vi "UHR-Fleezers Control (host) - Avogadro v1.vi"() -> ()   [LabVIEW 2014] (continued)
      }
      event "Green Laser ON/OFF", "Red Laser ON/OFF", "Blue Laser ON/OFF": Value Change {
        # "This loop shouldn't be initialized.  The main 'laser ON' settings should dominate and set the others."
        n1323 = event-data() -> ()  [unwired: 7 out]
        n1324 = property on="Red Laser ON" class="Bool (strict)"("Val(Sgnl)"="Red Laser ON/OFF") -> ()  [unwired: 2 in, 2 out]
        n1325 = property on="Blue Laser ON" class="Bool (strict)"("Val(Sgnl)"="Blue Laser ON/OFF") -> ()  [unwired: 2 in, 2 out]
        n1326 = property on="Green Laser ON" class="Bool (strict)"("Val(Sgnl)"="Green Laser ON/OFF") -> ()  [unwired: 2 in, 2 out]
      }
      event "Laser interlacing mode", "Green Laser ON", "Red Laser ON", "Blue Laser ON": Value Change {
        n1327 = event-data() -> ()  [unwired: 7 out]
        n1328 = local write "Green Laser ON/OFF"("Green Laser ON") -> ()
        n1329 = local write "Blue Laser ON/OFF"("Blue Laser ON") -> ()
        n1330 = local write "Red Laser ON/OFF"("Red Laser ON") -> ()
        n1331 = case shown="False" "Green Laser ON" {
          tunnel: "Laser interlacing mode" -> [_ w2112]
          tunnel: [enum32{"Laser ON", "Laser OFF", "Interlace"}."Laser OFF" ("Green laser mode") w2112] -> w2088
          tunnel: [FALSE w2108] -> w2087
          frame False {
          }
          frame True {
            n1332 = local read "Green FB On/Off"() -> (w2109:bool)
            n1333 = Equal?(x=w2112, y=enum32{"Laser ON", "Laser OFF", "Interlace"}."Interlace") -> (x = y?=w2110:bool)
            n1334 = And(x=w2110, y=w2109) -> (x .and. y?=w2108:bool)
          }
        }
        n1335 = case shown="True" "Red Laser ON" {
          tunnel: "Laser interlacing mode" -> [_ w2105]
          tunnel: [enum32{"Laser ON", "Laser OFF", "Interlace"}."Laser OFF" ("Green laser mode") w2105] -> w2084
          tunnel: [FALSE w2101] -> w2083
          frame False {
          }
          frame True {
            n1336 = local read "Red FB On/Off"() -> (w2102:bool)
            n1337 = Equal?(x=w2105, y=enum32{"Laser ON", "Laser OFF", "Interlace"}."Interlace") -> (x = y?=w2103:bool)
            n1338 = And(x=w2103, y=w2102) -> (x .and. y?=w2101:bool)
          }
        }
        n1339 = case shown="True" "Blue Laser ON" {
          tunnel: "Laser interlacing mode" -> [_ w2096]
          tunnel: [enum32{"Laser ON", "Laser OFF", "Interlace"}."Laser OFF" ("Green laser mode") w2096] -> w2080
          tunnel: [FALSE w2094] -> w2079
          frame False {
          }
          frame True {
            n1340 = local read "Blue FB On/Off"() -> (w2095:bool)
            n1341 = Equal?(x=w2096, y=enum32{"Laser ON", "Laser OFF", "Interlace"}."Interlace") -> (x = y?=w2097:bool)
            n1342 = And(x=w2097, y=w2095) -> (x .and. y?=w2094:bool)
          }
        }
        n1343 = xnode "Read/Write Control"("FPGA VI Reference In"=w2078, "Operating Mode"=w2088, "Operating Mode 2"=w2088, "Green FB On/Off"=w2087, "Red Laser Operating Mode"=w2084, "RI Operating Mode 2"=w2084, "Red FB On/Off"=w2083, "BI Operating Mode (AO)"=w2080, "Blue Laser Operating Mode (D)"=w2080, "Blue FB On/Off"=w2079) -> ("error out"=w2089:errorcluster)  [unwired: 1 in, 1 out]
        n1344 = local read "Red FB On/Off"() -> (w2061:bool)
        n1345 = local read "Green FB On/Off"() -> (w2063:bool)
        n1346 = local read "Green Laser ON"() -> (w2062:bool)
        n1347 = local read "Red Laser ON"() -> (w2060:bool)
        n1348 = And(x=w2061, y=w2060) -> (x .and. y?=w2066:bool)
        n1349 = And(x=w2063, y=w2062) -> (x .and. y?=w2072:bool)
        n1350 = local read "Red laser intensity (V)"() -> (w2065:dbl)
        n1351 = local read "Red FB Setpoint (mV)"() -> (w2064:dbl)
        n1352 = local read "Green FB Setpoint (mV)"() -> (w2075:dbl)
        n1353 = local read "Green laser intensity (V)"() -> (w2077:dbl)
        n1354 = Multiply(x=w2065, y=1000.0) -> (x*y=w2069:dbl)
        n1355 = Subtract(x=w2064, y=5.0) -> (x-y=w2068:dbl)
        n1356 = Multiply(x=w2077, y=1000.0) -> (x*y=w2074:dbl)
        n1357 = Subtract(x=w2075, y=5.0) -> (x-y=w2073:dbl)
        n1358 = Less Or Equal?(x=w2069, y=w2068) -> (x <= y?=w2067:bool)
        n1359 = Less Or Equal?(x=w2074, y=w2073) -> (x <= y?=w2071:bool)
        n1360 = And(x=w2066, y=w2067) -> (x .and. y?=w2056:bool)
        n1361 = And(x=w2072, y=w2071) -> (x .and. y?=w2057:bool)
        n1362 = Or(x=w2057, y=w2056) -> (x .or. y?=w2055:bool)
        n1363 = case shown="True" w2055 {
          frame False {
            n1364 = local write "Laser Intensity Low (bugs to fix)"(FALSE ("Laser Intensity Low")) -> ()
          }
          frame True {
            n1365 = local write "Laser Intensity Low (bugs to fix)"(TRUE ("Laser Intensity Low")) -> ()
          }
        }
      }
      event "Invert laser interlacing": Value Change {
        n1366 = event-data() -> ()  [unwired: 7 out]
        n1367 = xnode "Read/Write Control"("FPGA VI Reference In"=w2113, "Invert GI"="Invert laser interlacing", "Invert GI 2"="Invert laser interlacing", "Invert RI"="Invert laser interlacing", "Invert RI 2"="Invert laser interlacing", "Invert BI (AO)"="Invert laser interlacing", "Invert BI (D)"="Invert laser interlacing") -> ("error out"=w2115:errorcluster)  [unwired: 1 in, 1 out]
      }
      event "Green FB Setpoint (mV)", "Green FB Gains", "Green FB On/Off", "Green Intensity % (FB OFF)", "Green int current ON count adj": Value Change {
        n1368 = event-data() -> ()  [unwired: 7 out]
        n1369 = local read "Green FB Setpoint (mV)"() -> (w2135:dbl)
        n1370 = Multiply(x=w2135, y=3.2767) -> (x*y=w2134:dbl)
        n1371 = local read "Green Intensity % (FB OFF)"() -> (w2138:dbl)
        n1372 = Multiply(x=w2138, y=655.35) -> (x*y=w2139:dbl)
        n1373 = To Unsigned Word Integer(number=w2139) -> (unsigned 16bit integer=w2137:u16)
        n1374 = local read "Green int current ON count adj"() -> (w2141:u32)
        n1375 = local read "Laser interlacing mode"() -> (w2132:enum32{"Laser ON", "Laser OFF", "Interlace"})
        n1376 = local read "Green FB Gains"() -> (w2129:T14)
        n1377 = local read "Green Laser ON"() -> (w2133:bool)
        n1378 = local read "Green FB On/Off"() -> (w2142:bool)
        n1379 = Equal?(x=w2132, y=enum32{"Laser ON", "Laser OFF", "Interlace"}."Interlace") -> (x = y?=w2130:bool)
        n1380 = Unbundle By Name(w2129) -> ("proportional gain (Kc)"=w2128:i16, "integral gain (Kc*Ts/Ti)"=w2127:i16, "derivative gain (Kc*Td/Ts)"=w2126:i16)
        n1381 = Compound Arithmetic op=AND(w2130, w2142, w2133) -> (w2116:bool)
        n1382 = local read "Green FB Setpoint (mV)"() -> (w2120:dbl)
        n1383 = local read "Green laser intensity (V)"() -> (w2123:dbl)
        n1384 = xnode "Read/Write Control"("FPGA VI Reference In"=w2125, "Green FB Setpoint"=w2134, "Green FB On/Off"=w2116, "Current Out"=w2137, "Green int current ON count adj"=w2141, "P3"=w2128, "I3"=w2127, "D3"=w2126) -> ("error out"=w2143:errorcluster)  [unwired: 1 in, 1 out]
        n1385 = Multiply(x=w2123, y=1000.0) -> (x*y=w2119:dbl)
        n1386 = Subtract(x=w2120, y=5.0) -> (x-y=w2118:dbl)
        n1387 = Less Or Equal?(x=w2119, y=w2118) -> (x <= y?=w2117:bool)
        n1388 = And(x=w2116, y=w2117) -> (x .and. y?=w2124:bool)
        n1389 = case shown="True" w2124 {
          frame False {
            n1390 = local write "Laser Intensity Low (bugs to fix)"(FALSE ("Laser Intensity Low")) -> ()
          }
          frame True {
            n1391 = local write "Laser Intensity Low (bugs to fix)"(TRUE ("Laser Intensity Low")) -> ()
          }
        }
      }
      event "Blue FB Setpoint (mV)", "Blue FB Gains", "Blue FB On/Off", "Blue Intensity % (FB OFF)", "Blue int AO ON count adjust": Value Change {
        # "Triggers blue laser serial command"
        # "16 bit analog out"
        n1392 = event-data() -> ()  [unwired: 7 out]
        n1393 = Multiply(x="Blue FB Setpoint (mV)", y=3.2767) -> (x*y=w2163:dbl)
        n1394 = Multiply(x="Blue Intensity % (FB OFF)", y=0.8) -> (x*y=w2146:dbl)
        n1395 = Number To Decimal String(number=w2146) -> (decimal integer string=w2147:string)  [unwired: 1 in]
        n1396 = Multiply(x="Blue Intensity % (FB OFF)", y=655.35) -> (x*y=w2166:dbl)
        n1397 = local write "Blue Laser Power (mW)\n(Constant Power Mode)"(w2147) -> ()
        n1398 = To Unsigned Word Integer(number=w2166) -> (unsigned 16bit integer=w2165:u16)
        n1399 = local read "Laser interlacing mode"() -> (w2161:enum32{"Laser ON", "Laser OFF", "Interlace"})
        n1400 = Unbundle By Name("Blue FB Gains") -> ("proportional gain (Kc)"=w2158:i16, "integral gain (Kc*Ts/Ti)"=w2157:i16, "derivative gain (Kc*Td/Ts)"=w2156:i16)
        n1401 = local read "Blue Laser ON"() -> (w2151:bool)
        n1402 = Equal?(x=w2161, y=enum32{"Laser ON", "Laser OFF", "Interlace"}."Interlace") -> (x = y?=w2159:bool)
        n1403 = Compound Arithmetic op=AND(w2159, "Blue FB On/Off", w2151) -> (w2162:bool)
        n1404 = xnode "Read/Write Control"("FPGA VI Reference In"=w2150, "Blue FB Setpoint"=w2163, "Blue FB On/Off"=w2162, "BI Current Out"=w2165, "Blue current ON count adj (AO)"="Blue int AO ON count adjust", "P5"=w2158, "I5"=w2157, "D5"=w2156) -> ("error out"=w2168:errorcluster)  [unwired: 1 in, 1 out]
      }
      event "Red FB Setpoint (mV)", "Red FB Gains", "Red FB On/Off", "Red Intensity % (FB OFF)": Value Change {
        n1405 = event-data() -> ()  [unwired: 7 out]
        n1406 = local read "Red FB Setpoint (mV)"() -> (w2189:dbl)
        n1407 = Multiply(x=w2189, y=3.2767) -> (x*y=w2188:dbl)
        n1408 = local read "Red Intensity % (FB OFF)"() -> (w2179:dbl)
        n1409 = Multiply(x=w2179, y=655.35) -> (x*y=w2192:dbl)
        n1410 = To Unsigned Word Integer(number=w2192) -> (unsigned 16bit integer=w2191:u16)
        n1411 = local read "Laser interlacing mode"() -> (w2186:enum32{"Laser ON", "Laser OFF", "Interlace"})
        n1412 = local read "Red FB Gains"() -> (w2183:T14)
        n1413 = local read "Red Laser ON"() -> (w2187:bool)
        n1414 = local read "Red FB On/Off"() -> (w2194:bool)
        n1415 = Equal?(x=w2186, y=enum32{"Laser ON", "Laser OFF", "Interlace"}."Interlace") -> (x = y?=w2184:bool)
        n1416 = Unbundle By Name(w2183) -> ("proportional gain (Kc)"=w2182:i16, "integral gain (Kc*Ts/Ti)"=w2181:i16, "derivative gain (Kc*Td/Ts)"=w2180:i16)
        n1417 = Compound Arithmetic op=AND(w2184, w2194, w2187) -> (w2171:bool)
        n1418 = local read "Red laser intensity (V)"() -> (w2170:dbl)
        n1419 = local read "Red FB Setpoint (mV)"() -> (w2169:dbl)
        n1420 = xnode "Read/Write Control"("FPGA VI Reference In"=w2178, "Red FB Setpoint"=w2188, "Red FB On/Off"=w2171, "RI Current Out"=w2191, "P4"=w2182, "I4"=w2181, "D4"=w2180) -> ("error out"=w2195:errorcluster)  [unwired: 1 in, 1 out]
        n1421 = Multiply(x=w2170, y=1000.0) -> (x*y=w2175:dbl)
        n1422 = Subtract(x=w2169, y=5.0) -> (x-y=w2174:dbl)
        n1423 = Less Or Equal?(x=w2175, y=w2174) -> (x <= y?=w2173:bool)
        n1424 = And(x=w2171, y=w2173) -> (x .and. y?=w2172:bool)
        n1425 = case shown="False" w2172 {
          frame False {
            n1426 = local write "Laser Intensity Low (bugs to fix)"(FALSE ("Laser Intensity Low")) -> ()
          }
          frame True {
            n1427 = local write "Laser Intensity Low (bugs to fix)"(TRUE ("Laser Intensity Low")) -> ()
          }
        }
      }
      event "+ phase (APD 1 Gate)", "- phase (APD 1 Gate)", "+ phase (APD 2 Gate)", "- phase (APD 2 Gate)", "+ phase (APD 3 Gate)", "- phase (APD 3 Gate)", "+ phase (APD Acq)", "- phase (APD Acq)": Value Change {
        n1428 = event-data() -> ()  [unwired: 7 out]
        n1429 = local read "Phase Adj. (APD 1 Gate)"() -> (w2218:i16)
        n1430 = Or(x="- phase (APD 1 Gate)", y="+ phase (APD 1 Gate)") -> (x .or. y?=w2220:bool)
        n1431 = Negate(x=w2218) -> (-x=w2225:i16)
        n1432 = Select(t=w2225, s="+ phase (APD 1 Gate)", f=w2218) -> (s? t:f=w2224:i16)
        n1433 = local read "Phase Adj. (APD 2 Gate)"() -> (w2215:i16)
        n1434 = Or(x="- phase (APD 2 Gate)", y="+ phase (APD 2 Gate)") -> (x .or. y?=w2213:bool)
        n1435 = Negate(x=w2215) -> (-x=w2217:i16)
        n1436 = Select(t=w2217, s="+ phase (APD 2 Gate)", f=w2215) -> (s? t:f=w2214:i16)
        n1437 = Negate(x="Phase Adj. (APD 3 Gate)") -> (-x=w2212:i16)
        n1438 = Or(x="- phase (APD 3 Gate)", y="+ phase (APD 3 Gate)") -> (x .or. y?=w2208:bool)
        n1439 = Select(t=w2212, s="+ phase (APD 3 Gate)", f="Phase Adj. (APD 3 Gate)") -> (s? t:f=w2209:i16)
        n1440 = local read "Phase Adj. (APD Acq)"() -> (w2206:i16)
        n1441 = Or(x="- phase (APD Acq)", y="+ phase (APD Acq)") -> (x .or. y?=w2204:bool)
        n1442 = Negate(x=w2206) -> (-x=w2207:i16)
        n1443 = Select(t=w2207, s="+ phase (APD Acq)", f=w2206) -> (s? t:f=w2205:i16)
        n1444 = xnode "Read/Write Control"("FPGA VI Reference In"=w2198, "Phase count adjustment (APD 1 Gate)"=w2224, "Phase count adjustment (APD 2 Gate)"=w2214, "Phase count adjustment (APD 3 Gate)"=w2209, "Phase Count Adjustment (APD Acq)"=w2205) -> ("FPGA VI Reference Out"=w2222:T41, "error out"=w2223:errorcluster)  [unwired: 1 in]
        n1445 = xnode "Read/Write Control"("FPGA VI Reference In"=w2222, "error in"=w2223, "+ phase (APD 1 Gate)"=w2220, "+ phase (APD 2 Gate)"=w2213, "+ phase (APD 3 Gate)"=w2208, "+ phase (APD Acq)"=w2204) -> ("error out"=w2221:errorcluster)  [unwired: 1 out]
      }
      event "Invert APD Gate", "APD Gate ON Count", "APD Gate OFF Count", "APD Gate", "APD Integration Time (s)", "APD AO Scale Factor", "Duty Frequency (ON 1/N cycles)", "Interlace ON count", "Interlace OFF count": Value Change {
        n1446 = event-data() -> ()  [unwired: 7 out]
        n1447 = Add(x="Interlace ON count", y="Interlace OFF count") -> (x+y=w2232:u16)
        n1448 = Add(x="APD Gate ON Count", y="APD Gate OFF Count") -> (x+y=w2243:u16)
        n1449 = Multiply(x="Duty Frequency (ON 1/N cycles)", y=w2232) -> (x*y=w2228:u16)
        "Green AI Count" <- w2228
        "Red AI Count" <- w2228
        "Blue AI Count" <- w2228
        n1450 = Subtract(x=w2228, y="Interlace ON count") -> (x-y=w2231:u16)
        n1451 = Multiply(x=w2243, y="Duty Frequency (ON 1/N cycles)") -> (x*y=w2242:u16)
        n1452 = Subtract(x=w2242, y="APD Gate ON Count") -> (x-y=w2241:u16)
        n1453 = local read "DMA Update Period (s)"() -> (w2244:dbl)
        n1454 = Multiply(x="APD Integration Time (s)", y=40000000.0) -> (x*y=w2248:dbl)
        n1455 = Reciprocal(x="APD Integration Time (s)") -> (1/x=→"APD Acq Rate (Hz)":dbl)
        n1456 = To Unsigned Long Integer(number=w2248) -> (unsigned 32bit integer=w2234:u32)
        "APD Int. Count" <- w2234
        n1457 = local read "Number of APDs"() -> (w2227:u8)
        n1458 = Divide(x=w2244, y="APD Integration Time (s)") -> (x/y=w2246:dbl)
        n1459 = Multiply(x=w2227, y=w2246) -> (x*y=w2245:dbl)
        n1460 = local write "APD Samples/FIFO Acq."(w2246) -> ()
        n1461 = local write "APD Elements/DMA read"(w2245) -> ()
        n1462 = xnode "Read/Write Control"("FPGA VI Reference In"=w2226, "Invert APD Gate"="Invert APD Gate", "APD Gate ON Count"="APD Gate ON Count", "APD Gate OFF Count"=w2241, "APD Acq Rate Count"=w2234, "APD Gate Operating Mode"="APD Gate", "APD AO scale factor"="APD AO Scale Factor", "Green interlace ON count"="Interlace ON count", "Green interlace OFF count"=w2231, "Green interlace ON count 2"="Interlace ON count", "Green interlace OFF count 2"=w2231, "Green FB Count"=w2228, "Red interlace ON count"="Interlace ON count", "Red interlace OFF count"="Interlace OFF count", "Blue ON count (AO)"="Interlace ON count", "Blue OFF count (AO)"="Interlace OFF count", "Blue interlace OFF count (D)"="Interlace OFF count", "Blue interlace ON count (D)"="Interlace ON count") -> ("error out"=w2250:errorcluster)  [unwired: 1 in, 1 out]
      }
      event "Neg. TTrig FPGA": Value Change {
        n1463 = event-data() -> ()  [unwired: 7 out]
        n1464 = xnode "Read/Write Control"("FPGA VI Reference In"=w2251, "TTrig Negate Pos"="Neg. TTrig FPGA") -> ()  [unwired: 1 in, 2 out]
      }
      event "Test ttrig": Value Change {
        n1465 = event-data() -> ()  [unwired: 7 out]
        n1466 = xnode "Read/Write Control"("FPGA VI Reference In"=w2253, "TTrig?"=TRUE) -> ("error out"=w2255:errorcluster)  [unwired: 1 in, 1 out]
      }
      event "Number of F/B Scans (AOD)", "Scan Speed (nm/s)", "Scan BD", "Initial delta (MHz)", "Step Size (nm)", "Scan Range (nm)": Value Change {
        w2319 = 123.0  # AOM cal (nm/MHz)
        n1467 = event-data() -> ()  [unwired: 7 out]
        n1468 = local read "BD 1 Frequency 1 (MHz)"() -> (w2302:dbl)
        n1469 = local read "AOM X Cal (nm/MHz)"() -> (w2294:dbl)
        n1470 = local read "X RF Frequency Limits (MHz)"() -> (w2306:T23)
        n1471 = local read "Y RF Frequency Limits (MHz)"() -> (w2303:T23)
        n1472 = local read "BD 2 Frequency 1 (MHz)"() -> (w2308:dbl)
        n1473 = Negate(x="Scan Range (nm)") -> (-x=w2272:dbl)
        n1474 = Divide(x=w2272, y=w2294) -> (x/y=w2276:dbl)
        n1475 = Select(t=w2306, s="Scan BD", f=w2303) -> (s? t:f=w2305:T23)
        n1476 = Select(t=w2302, s="Scan BD", f=w2308) -> (s? t:f=w2307:dbl)
        n1477 = Unbundle By Name(w2305) -> ("Maximum"=w2314:dbl, "Minimum"=w2313:dbl)
        n1478 = Add(x=w2276, y=w2307) -> (x+y=w2311:dbl)
        n1479 = Divide(x=w2272, y="Step Size (nm)") -> (x/y=w2291:dbl)
        n1480 = Divide(x="Step Size (nm)", y=w2294) -> (x/y=w2300:dbl)
        n1481 = Absolute Value(x=w2291) -> (abs(x)=w2275:dbl)
        n1482 = Sign(1:w2272) -> (0:w2273:dbl)
        n1483 = In Range and Coerce(upper limit=w2314, x=w2311, lower limit=w2313) -> (coerced(x)=w2310:dbl, In Range?=w2312:bool)
        n1484 = To Unsigned Quad Integer(1:w2275) -> (0:w2290:u64)
        "Scan steps (AOD)" <- w2290
        n1485 = call "IR AOM freq to word.vi"("Frequency In (MHz)"=w2300) -> ("Frequency Word Out (double)"=w2297:dbl)
        n1486 = Multiply(x=w2273, y=w2297) -> (x*y=w2274:dbl)
        n1487 = Subtract(x=w2311, y=w2310) -> (x-y=w2309:dbl)
        n1488 = To Quad Integer(1:w2274) -> (0:w2296:i64)
        "Incr. int (AOD)" <- w2296
        n1489 = Subtract(x=w2276, y=w2309) -> (x-y=w2295:dbl)
        "Scan Range (MHz)" <- w2295
        n1490 = Select(t=w2276, s=w2312, f=w2295) -> (s? t:f=w2315:dbl)
        n1491 = Multiply(x=w2295, y=w2294) -> (x*y=w2293:dbl)
        n1492 = Decrement(x=w2290) -> (x-1=w2343:u64)
        n1493 = Negate(x=w2293) -> (-x=w2289:dbl)
        n1494 = local write "Scan Range (nm)"(w2289) -> ()
        n1495 = Divide(x=w2315, y=w2343) -> (x/y=w2299:dbl)
        "Scan Increment (MHz)" <- w2299
        n1496 = call "IR AOM freq to word.vi"("Frequency In (MHz)"=w2299) -> ("Frequency Word Out (double)"=w2298:dbl)
        n1497 = Divide(x="Step Size (nm)", y="Scan Speed (nm/s)") -> (x/y=w2286:dbl)
        n1498 = To Quad Integer(1:w2298) -> ()  [unwired: 1 out]
        n1499 = local read "Number Interlace Sets"() -> (w2270:u8)
        n1500 = local read "AI Count (ticks)"() -> (w2271:u16)
        n1501 = local read "Total Counts (ticks)"() -> (w2269:u16)
        n1502 = local read "# Samples/trap"() -> (w2301:u32)
        n1503 = Multiply(x=w2271, y=w2270) -> (x*y=w2268:u16)
        n1504 = Divide(x=w2269, y=w2268) -> (x/y=w2267:dbl)
        n1505 = Select(t=w2302, s="Scan BD", f=w2308) -> (s? t:f=w2340:dbl)
        "Initial freq. (MHz)" <- w2340
        n1506 = Add(x=w2315, y=w2340) -> (x+y=→"Final freq. (MHz)":dbl)
        n1507 = Divide(x=w2269, y=40000000.0) -> (x/y=w2285:dbl)
        n1508 = Divide(x=w2286, y=w2285) -> (x/y=w2284:dbl)
        n1509 = To Unsigned Quad Integer(1:w2284) -> (0:w2259:u64)
        n1510 = Quotient & Remainder(x=w2259, y=u64 2) -> (x-y*floor(x/y)=w2263:u64)  [unwired: 1 out]
        n1511 = Equal?(x=w2263, y=u64 0) -> (x = y?=w2261:bool)
        n1512 = Decrement(x=w2259) -> (x-1=w2260:u64)
        n1513 = Select(t=w2259, s=w2261, f=w2260) -> (s? t:f=w2258:u64)
        "Cycles/step (AOD)" <- w2258
        n1514 = xnode "Read/Write Control"("FPGA VI Reference In"=w2257, "Scan steps"=w2290, "Number of scans"="Number of F/B Scans (AOD)", "Cycles per step"=w2258, "Scan freq.  increment"=w2296, "Scan BD"="Scan BD") -> ("error out"=w2349:errorcluster)  [unwired: 1 in, 1 out]
        n1515 = Multiply(x=w2290, y=w2258) -> (x*y=w2344:u64)
        n1516 = Multiply(x=w2344, y=u64 2) -> (x*y=w2266:u64)
        n1517 = Multiply(x=w2267, y=w2266) -> (x*y=w2265:dbl)
        "Data points/scan (f/b)" <- w2265
        n1518 = Multiply(x=w2265, y="Number of F/B Scans (AOD)") -> (x*y=w2347:dbl)
        "Data points/scans" <- w2347
        n1519 = Divide(x=w2347, y=w2301) -> (x/y=→"N sets should be saved":dbl)
        n1520 = Multiply(x=w2344, y=w2285) -> (x*y=w2283:dbl)
        "Time/Scan (s) (AOD)" <- w2283
        n1521 = Select(t=w2315, s="Scan BD", f=0.0) -> (s? t:f=w2341:dbl)
        n1522 = Select(t=0.0, s="Scan BD", f=w2315) -> (s? t:f=w2337:dbl)
        n1523 = local read "BD 2 Frequency 2 (MHz)"() -> (w2333:dbl)
        n1524 = local read "BD 1 Frequency 2 (MHz)"() -> (w2336:dbl)
        n1525 = Add(x=w2337, y=w2308) -> (x+y=w2334:dbl)
        n1526 = Add(x=w2302, y=w2341) -> (x+y=w2335:dbl)
        n1527 = Multiply(x=w2283, y=2.0) -> (x*y=w2282:dbl)
        n1528 = Multiply(x=w2282, y="Number of F/B Scans (AOD)") -> (x*y=w2279:dbl)
        n1529 = Divide(x=w2279, y=60.0) -> (x/y=→"Time to Finish All (min)":dbl)
        n1530 = Add(x="Trap 2 Bead Size (nm)", y="Trap 1 Bead Size (nm)") -> (x+y=w2323:dbl)
        n1531 = Divide(x=w2323, y=2.0) -> (x/y=w2317:dbl)
        n1532 = local read "Initial delta (MHz)"() -> (w2320:dbl)
        n1533 = Subtract(x=w2334, y=w2333) -> (x-y=w2331:dbl)
        n1534 = Subtract(x=w2335, y=w2336) -> (x-y=w2332:dbl)
        n1535 = Square(x=w2331) -> (x^2=w2330:dbl)
        n1536 = Square(x=w2332) -> (x^2=w2329:dbl)
        n1537 = Add(x=w2329, y=w2330) -> (x+y=w2328:dbl)
        n1538 = Square Root(x=w2328) -> (sqrt(x)=w2327:dbl)
        "Final delta (MHz)" <- w2327
        n1539 = Multiply(x=w2319, y=w2327) -> (x*y=w2326:dbl)
        n1540 = Multiply(x=w2320, y=w2319) -> (x*y=w2318:dbl)
        n1541 = Subtract(x=w2318, y=w2317) -> (x-y=→"Initial sep (nm)":dbl)
        n1542 = Subtract(x=w2326, y=w2317) -> (x-y=→"Final sep (nm)":dbl)
      }
      event "Freq or Amp switch first", "Swap F1 and F2", "Freq switch delay", "Amp switch delay": Value Change {
        n1543 = event-data() -> ()  [unwired: 7 out]
        n1544 = local read "Amp switch delay"() -> (w2351:u16)
        n1545 = local read "Swap F1 and F2"() -> (w2352:bool)
        n1546 = xnode "Read/Write Control"("FPGA VI Reference In"=w2350, "Swap F1 and F2"=w2352, "Amp switch delay"=w2351) -> ("error out"=w2353:errorcluster)  [unwired: 1 in, 1 out]
      }
      event "Scan steps (MCL)", "Number of scans (MCL)", "Scan Range (V)\n(of steps)", "2D or 1D Scan", "N APD Samp/step", "Fast Scan Dir", "Continuous MCL Scanning", "Scan lines (y)": Value Change {
        w2356 = 32767.0 ("y")
        n1547 = event-data() -> ()  [unwired: 7 out]
        n1548 = Select(t="Scan lines (y)", s="2D or 1D Scan", f="Number of scans (MCL)") -> (s? t:f=w2361:u64)
        n1549 = Decrement(x="Scan steps (MCL)") -> (x-1=w2377:u64)
        n1550 = Divide(x="Scan Range (V)\n(of steps)", y=w2377) -> (x/y=w2376:dbl)
        "Desired Scan Incr (V)" <- w2376
        n1551 = local read "APD Integration Time (s)"() -> (w2369:dbl)
        n1552 = Multiply(x=w2376, y=w2356) -> (x*y=w2385:dbl)
        n1553 = Divide(x=w2385, y=10.0) -> (x/y=w2375:dbl)
        "Desired incr (int)" <- w2375
        n1554 = local read "Update Count (MCL)"() -> (w2381:u32)
        n1555 = Round Toward -Infinity(1:w2375) -> (0:w2384:dbl)
        n1556 = To Word Integer(number=w2384) -> (16bit integer=w2359:i16)
        "Actual Incr. int (MCL)" <- w2359
        n1557 = Multiply(x=w2369, y=40000000.0) -> (x*y=w2382:dbl)
        n1558 = Divide(x=w2382, y=w2381) -> (x/y=w2380:dbl)
        n1559 = Multiply(x=i16 10, y=w2359) -> (x*y=w2357:i16)
        n1560 = Multiply(x="N APD Samp/step", y=w2380) -> (x*y=w2379:dbl)
        "Cycles/step (MCL)" <- w2379
        n1561 = Divide(x=w2357, y=w2356) -> (x/y=→"Actual MCL Inc (V)":dbl)
        n1562 = Multiply(x="N APD Samp/step", y="Scan steps (MCL)") -> (x*y=w2371:dbl)
        n1563 = local read "APD Samples/FIFO Acq."() -> (w2368:dbl)
        n1564 = Multiply(x=w2371, y=u64 2) -> (x*y=w2370:dbl)
        "Data points/scan (f+b)" <- w2370
        n1565 = Multiply(x=w2370, y=w2361) -> (x*y=w2388:dbl)
        "Data points/scans (MCL)" <- w2388
        n1566 = Multiply(x=w2369, y=w2370) -> (x*y=w2362:dbl)
        "Time/f+b scan (s) (MCL)" <- w2362
        n1567 = Divide(x=w2388, y=w2368) -> (x/y=→"N sets should be saved (MCL)":dbl)
        n1568 = Multiply(x=w2362, y=w2361) -> (x*y=→"Total Time (s)":dbl)
        n1569 = Not(x="Fast Scan Dir") -> (.not. x?=w2366:bool)
        n1570 = xnode "Read/Write Control"("FPGA VI Reference In"=w2354, "Scan steps (MCL)"="Scan steps (MCL)", "Number of scans (MCL)"=w2361, "Cycles per step (MCL)"=w2379, "Scan freq.  increment (MCL)"=w2359, "1D or 2D Scan?"="2D or 1D Scan", "MCL Scan Axis"=w2366, "Cont. Scan (MCL)"="Continuous MCL Scanning") -> ("error out"=w2390:errorcluster)  [unwired: 1 in, 1 out]
      }
      event "Read Cal": Value Change {
        w2411 = T45."big-endian, network order" ("byte order (0:big-endian, network order)")
        n1571 = event-data() -> ()  [unwired: 7 out]
        n1572 = local read "Save file name"() -> (w2443:path)
        n1573 = Strip Path(path=w2443) -> (stripped path=w2442:path)  [unwired: 1 out]
        n1574 = Path To String(path=w2442) -> (string=w2435:string)
        n1575 = Concatenate Strings(w2435, "\\current.cal" ("string")) -> (w2440:string)
        n1576 = String To Path(string=w2440) -> (path=w2439:path)
        n1577 = Open/Create/Replace File(file path (use dialog)=w2439, operation (0:open)=T44."open", access (0:read/write)=enum16{"read/write", "read-only", "write-only"}."read-only") -> (refnum out=w2446:refnum<file>, error out=w2438:errorcluster)  [unwired: 1 in, 3 out]
        n1578 = Concatenate Strings(w2435, "\\current.off" ("string")) -> (w2433:string)
        n1579 = Deny Access(4:w2438, 7:w2446) -> (0:w2412:errorcluster, 3:w2407:refnum<file>)  [unwired: 1 out]
        n1580 = String To Path(string=w2433) -> (path=w2430:path)
        n1581 = local write "Read Cal"(FALSE ("Read Cal")) -> ()
        n1582 = Open/Create/Replace File(file path (use dialog)=w2430, operation (0:open)=T44."open", access (0:read/write)=enum16{"read/write", "read-only", "write-only"}."read-only") -> (refnum out=w2429:refnum<file>)  [unwired: 1 in, 4 out]
        n1583 = Deny Access(7:w2429) -> (3:w2428:refnum<file>)  [unwired: 1 in, 2 out]
        n1584 = Read from Binary File(5:0.0, 9:w2411, 10:-1 ("count (1)"), 11:w2428) -> (2:w2423:dbl[], 3:w2421:refnum<file>)  [unwired: 1 in, 3 out]
        n1585 = Close File(refnum=w2421) -> ()  [unwired: 1 in, 2 out]
        n1586 = Index Array(array=w2423, index=0) -> (element=→"Offset file step size":dbl)
        n1587 = Array Subset(array=w2423, index=1) -> (w2420:dbl[])  [unwired: 1 in]
        n1588 = Decimate 1D Array(w2420) -> (w2416:dbl[], w2415:dbl[])  [unwired: 1 out]
        n1589 = Build Array("T1 calibration", "T2 calibration", "T3 calibration") -> (w2403:T47)
        n1590 = for {
          N: 3 ("count (1)") -> [_]
          tunnel: w2411 -> [w2464]
          shift-right: [w2462] -> w2409
          shift-left: w2412 -> [w2465]
          shift-right: [w2461] -> w2408
          shift-left: w2407 -> [w2460]
          tunnel: w2403 -> [w2459] mode=indexing
          tunnel: [w2452] -> w2402 mode=indexing
          i -> [w2453]
          w2451 = 1000.0
          n1591 = Read from Binary File(5:0.0, 8:w2465, 9:w2464, 10:6 ("count (1)"), 11:w2460) -> (0:w2462:errorcluster, 2:w2467:dbl[], 3:w2461:refnum<file>)  [unwired: 2 out]
          n1592 = Array To Cluster(array=w2467) -> (cluster=w2458:T48)
          n1593 = Unbundle(w2458) -> ("[0]"=w2457:dbl, "[1]"=w2456:dbl, "[2]"=w2449:dbl, "[3]"=w2455:dbl, "[4]"=w2454:dbl, "[5]"=w2450:dbl)
          n1594 = Multiply(x=w2451, y=w2450) -> (x*y=w2447:dbl)
          n1595 = Multiply(x=w2451, y=w2449) -> (x*y=w2448:dbl)
          n1596 = Bundle By Name(cluster=w2459, "alpha_x (nm/V)"=w2457, "kappa_x (pN/nm)"=w2456, "offset_x (mV)"=w2448, "alpha_y (nm/V)"=w2455, "kappa_y (pN/nm)"=w2454, "offset_y (mV)"=w2447) -> (w2452:T9)
          n1597 = case shown="2" w2453 {
            tunnel: w2452 -> [w2468 w2469 w2470]
            frame 0, Default {
              n1598 = local write "T1 calibration"(w2468) -> ()
            }
            frame 1 {
              n1599 = local write "T2 calibration"(w2469) -> ()
            }
            frame 2 {
              n1600 = local write "T3 calibration"(w2470) -> ()
            }
          }
        }
        n1601 = Bundle By Name(cluster="Offset Values", "Trap 1X offset"=w2416, "Trap 2X offset"=w2415) -> (w2418:T20)
        n1602 = local write "Offset Values"(w2418) -> ()
        n1603 = Index Array(array=w2402, index=1) -> (element=w2399:T9)
        n1604 = Index Array(array=w2402, index=0) -> (element=w2398:T9)
        n1605 = Unbundle By Name(w2399) -> ("alpha_x (nm/V)"=w2397:dbl, "kappa_x (pN/nm)"=w2396:dbl)
        n1606 = Unbundle By Name(w2398) -> ("alpha_x (nm/V)"=w2395:dbl, "kappa_x (pN/nm)"=w2394:dbl)
        n1607 = Close File(refnum=w2408, error in=w2409) -> (error out=→"Read cal error":errorcluster)  [unwired: 1 out]
        n1608 = Multiply(x=w2397, y=w2396) -> (x*y=w2393:dbl)
        n1609 = Multiply(x=w2395, y=w2394) -> (x*y=w2392:dbl)
        n1610 = Divide(x=w2393, y=w2392) -> (x/y=w2391:dbl)
        n1611 = property on="B factor" class="DigNum (strict)"("Val(Sgnl)"=w2391) -> ()  [unwired: 2 in, 2 out]
        n1612 = Multiply(x=w2415, y=w2391) -> (x*y=w2417:dbl[])
        n1613 = Subtract(x=w2416, y=w2417) -> (x-y=w2413:dbl[])
        n1614 = case shown="True" "Auto read offset correction" {
          tunnel: w2413 -> [_ w2471]
          frame False {
          }
          frame True {
            n1615 = property on="Setpoint offset\ncorrection values" class="Arr (strict)"("Val(Sgnl)"=w2471) -> ()  [unwired: 2 in, 2 out]
          }
        }
      }
      event "Abort MCL Scan": Value Change {
        n1616 = event-data() -> ()  [unwired: 7 out]
        n1617 = local write "MCL Scanning"(FALSE ("MCL Scanning")) -> ()
        n1618 = xnode "Read/Write Control"("FPGA VI Reference In"=w2472, "Abort scan (MCL)"="Abort MCL Scan") -> ("error out"=w2475:errorcluster)  [unwired: 1 in, 1 out]
      }
      event "Update Count (MCL)": Value Change {
        n1619 = event-data() -> ()  [unwired: 7 out]
        n1620 = xnode "Read/Write Control"("FPGA VI Reference In"=w2476, "MCL count"="Update Count (MCL)") -> ("error out"=w2478:errorcluster)  [unwired: 1 in, 1 out]
      }
      event "+ phase (MCL)", "- phase (MCL)": Value Change {
        n1621 = event-data() -> ()  [unwired: 7 out]
        n1622 = Or(x="- phase (MCL)", y="+ phase (MCL)") -> (x .or. y?=w2482:bool)
        n1623 = Negate(x="Phase adjust (MCL)") -> (-x=w2488:i16)
        n1624 = Select(t=w2488, s="+ phase (MCL)", f="Phase adjust (MCL)") -> (s? t:f=w2486:i16)
        n1625 = xnode "Read/Write Control"("FPGA VI Reference In"=w2479, "Phase count adjustment (MCL)"=w2486) -> ("FPGA VI Reference Out"=w2483:T41, "error out"=w2484:errorcluster)  [unwired: 1 in]
        n1626 = xnode "Read/Write Control"("FPGA VI Reference In"=w2483, "error in"=w2484, "+ phase (MCL)"=w2482) -> ("error out"=w2481:errorcluster)  [unwired: 1 out]
      }
      event "Abort AOD Scan": Value Change {
        n1627 = event-data() -> ()  [unwired: 7 out]
        n1628 = xnode "Read/Write Control"("FPGA VI Reference In"=w2489, "Abort scan"="Abort AOD Scan") -> ("error out"=w2491:errorcluster)  [unwired: 1 in, 1 out]
      }
      event "Continuous AOD Scanning": Value Change {
        n1629 = event-data() -> ()  [unwired: 7 out]
        n1630 = xnode "Read/Write Control"("FPGA VI Reference In"=w2492, "Cont. Scan"="Continuous AOD Scanning") -> ("error out"=w2494:errorcluster)  [unwired: 1 in, 1 out]
      }
      event "Index": Value Change {
        n1631 = event-data() -> ()  [unwired: 7 out]
        n1632 = call "Create new save file.vi"("Insert"="", "Ext"=".dat" ("string"), "Index In"="Index") -> ("Path Out"=→"Save file name":path, "Index Out"=w2495:dbl)
        "Save index" <- w2495
        n1633 = local write "Index"(w2495) -> ()
      }
      event "AO1", "AO2": Value Change {
        w2509 = 10.0 ("y")
        w2508 = 32767.0 ("y")
        n1634 = event-data() -> ()  [unwired: 7 out]
        n1635 = local read "AO2"() -> (w2507:dbl)
        n1636 = local read "AO1"() -> (w2504:dbl)
        n1637 = Multiply(x=w2504, y=w2508) -> (x*y=w2503:dbl)
        n1638 = Multiply(x=w2507, y=w2508) -> (x*y=w2506:dbl)
        n1639 = Divide(x=w2503, y=w2509) -> (x/y=w2502:dbl)
        n1640 = Divide(x=w2506, y=w2509) -> (x/y=w2505:dbl)
        n1641 = To Word Integer(number=w2502) -> (16bit integer=w2510:i16)
        n1642 = To Word Integer(number=w2505) -> (16bit integer=w2511:i16)
        n1643 = xnode "Read/Write Control"("FPGA VI Reference In"=w2500, "AO1 (Y)"=w2510, "AO2 (X)"=w2511) -> ("error out"=w2501:errorcluster)  [unwired: 1 in, 1 out]
      }
      event "Inject Pump 1": Value Change {
        n1644 = event-data() -> ()  [unwired: 7 out]
        n1645 = disable-structure shown="Disabled" {
          disable-tunnel: w2512 -> [w2513 _]
          frame Disabled {
            n1646 = local read "Use Harvard pumps\nfor beads (else Chemyx)"() -> (w2514:bool)
            n1647 = case shown="True" w2514 {
              tunnel: "Inject Pump 1" -> [w2518 w2559]
              tunnel: w2513 -> [_ w2560]
              frame False {
                n1648 = local read "Pump write delay (ms)"() -> (w2517:dbl)
                n1649 = local read "Chemyx Syringe Pump Serial Port"() -> (w2516:refnum<visa-resource-name>)
                n1650 = case shown="True" w2518 {
                  tunnel: w2517 -> [w2524 w2538]
                  tunnel: w2516 -> [w2521 w2537]
                  frame False {
                    n1651 = flat-sequence {
                      tunnel: w2521 -> [w2525]
                      tunnel: [w2525] -> w2522
                      tunnel: w2524 -> [_]
                      tunnel: [w2528] -> w2523
                      tunnel: w2522 -> [w2528]
                      tunnel: w2523 -> [w2529]
                      tunnel: [w2529] -> w2519
                      tunnel: [w2531] -> w2520
                      tunnel: w2519 -> [w2531]
                      tunnel: w2520 -> [w2533]
                      frame #0 {
                        n1652 = call "Write to pump.vi"("string"="enter pump1", "VISA resource name"=w2525) -> ()  [unwired: 1 out]
                      }
                      frame #1 {
                        n1653 = Wait (ms)(milliseconds to wait="Pump pause delay (ms)") -> ()  [unwired: 1 out]
                      }
                      frame #2 {
                        n1654 = call "Write to pump.vi"("string"="stop", "VISA resource name"=w2529) -> ()  [unwired: 1 out]
                      }
                      frame #3 {
                        n1655 = Wait (ms)(milliseconds to wait=u32 500) -> ()  [unwired: 1 out]
                      }
                      frame #4 {
                        n1656 = call "Write to pump.vi"("string"="stop", "VISA resource name"=w2533) -> ()  [unwired: 1 out]
                      }
                    }
                  }
                  frame True {
                    n1657 = flat-sequence {
                      tunnel: w2537 -> [w2547]
                      tunnel: w2538 -> [w2542]
                      tunnel: w2538 -> [w2549]
                      tunnel: w2537 -> [w2550]
                      tunnel: [w2550] -> w2535
                      tunnel: [w2552] -> w2536
                      tunnel: w2535 -> [w2552]
                      tunnel: w2536 -> [w2554]
                      frame #0 {
                        n1658 = local read "All Pump Parameters"() -> (w2541:T10)
                        n1659 = Unbundle By Name(w2541) -> ("Pump 1"=w2548:T49)
                        n1660 = call "Set pump parameters.vi"("Pump write delay (ms)"=w2542, "Volume (uL)"="Ch 1 Inject Volume (uL)", "Rate (uL/h)"="Ch 1 Inject Rate (ul/h)", "Units"=4.0, "Pump #"=1.0, "Pump Parameters In"=w2548, "VISA resource name"=w2547) -> ("Pump Parameters Out"=w2540:T49)  [unwired: 3 in]
                        n1661 = Bundle By Name(cluster=w2541, "Pump 1"=w2540) -> (w2539:T10)
                        n1662 = local write "All Pump Parameters"(w2539) -> ()
                      }
                      frame #1 {
                        n1663 = Wait (ms)(milliseconds to wait=w2549) -> ()  [unwired: 1 out]
                      }
                      frame #2 {
                        n1664 = call "Write to pump.vi"("string"="start", "VISA resource name"=w2550) -> ()  [unwired: 1 out]
                      }
                      frame #3 {
                        n1665 = Wait (ms)(milliseconds to wait=u32 500) -> ()  [unwired: 1 out]
                      }
                      frame #4 {
                        n1666 = call "Write to pump.vi"("string"="start", "VISA resource name"=w2554) -> ()  [unwired: 1 out]
                      }
                    }
                  }
                }
              }
              frame True {
                n1667 = case shown="False" w2559 {
                  tunnel: w2560 -> [w2572 w2582]
                  frame False {
                    n1668 = flat-sequence {
                      tunnel: w2572 -> [w2574]
                      frame #0 {
                        n1669 = local write "Flushing P1"(FALSE ("Flushing P1")) -> ()
                        n1670 = Concatenate Strings("stop" ("string"), "\r") -> (w2576:string)
                        n1671 = VISA Write(VISA resource name=w2574, write buffer=w2576) -> ()  [unwired: 1 in, 3 out]
                      }
                      frame #1 {
                        n1672 = property on="Clear Volume P1" class="Bool (strict)"("Val(Sgnl)"=TRUE ("Value (Signaling)")) -> ()  [unwired: 2 in, 2 out]
                      }
                    }
                  }
                  frame True {
                    n1673 = local read "Normal Flow Rate (ul/h) P1"() -> (w2580:dbl)
                    n1674 = Number To Decimal String(number=w2580) -> (decimal integer string=w2586:string)  [unwired: 1 in]
                    n1675 = Concatenate Strings("irate  " ("string"), w2586, " u/h" ("string"), "\r") -> (w2584:string)
                    n1676 = VISA Write(VISA resource name=w2582, write buffer=w2584) -> (VISA resource name out=w2581:refnum<visa-resource-name>)  [unwired: 1 in, 2 out]
                    n1677 = Concatenate Strings("irun" ("string"), "\r") -> (w2588:string)
                    n1678 = VISA Write(VISA resource name=w2581, write buffer=w2588) -> ()  [unwired: 1 in, 3 out]
                  }
                }
                n1679 = local read "Saving..."() -> (w2557:bool)
                n1680 = local read "Save Event Log?"() -> (w2556:bool)
                n1681 = And(x=w2557, y=w2556) -> (x .and. y?=w2558:bool)
                n1682 = case shown="True" w2558 {
                  tunnel: w2559 -> [_ w2570]
                  frame False {
                  }
                  frame True {
                    n1683 = local read "Normal Flow Rate (ul/h) P1"() -> (w2561:dbl)
                    n1684 = Number To Decimal String(number=w2561) -> (decimal integer string=w2562:string)  [unwired: 1 in]
                    n1685 = Concatenate Strings("on, flow rate", w2562) -> (w2564:string)
                    n1686 = Select(t=w2564, s=w2570, f="off") -> (s? t:f=w2566:string)
                    n1687 = local read "log file ref"() -> (w2571:refnum<file>)
                    n1688 = local read "Time (s)"() -> (w2565:dbl)
                    n1689 = Concatenate Strings("pump 1 ", w2566) -> (w2568:string)
                    n1690 = call "write to event log.vi"("log file ref"=w2571, "time"=w2565, "input string"=w2568) -> ()  [unwired: 8 in]
                  }
                }
              }
            }
          }
          frame Enabled {
          }
        }
      }
      event "Shunt 1": Value Change {
        n1691 = event-data() -> ()  [unwired: 7 out]
        n1692 = local read "Visa resource for valves"() -> (w2590:refnum<visa-resource-name>)
        n1693 = call "hamilton_controller.vi"("VISA resource name in"=w2590, "Open?"="Shunt 1", "valve"=enum16{"A", "B", "ALL"}."A", "action"=T42."MOVE VALVE") -> ("error out"=w2592:errorcluster)  [unwired: 6 in, 1 out]
      }
      event "Shunt 2": Value Change {
        n1694 = event-data() -> ()  [unwired: 7 out]
        n1695 = local read "Visa resource for valves"() -> (w2595:refnum<visa-resource-name>)
        n1696 = call "hamilton_controller.vi"("VISA resource name in"=w2595, "Open?"="Shunt 2", "valve"=enum16{"A", "B", "ALL"}."B", "action"=T42."MOVE VALVE") -> ("error out"=w2596:errorcluster)  [unwired: 6 in, 1 out]
      }
      event "Inject Pump 3": Value Change {
        n1697 = event-data() -> ()  [unwired: 7 out]
        n1698 = local read "Use Harvard pumps\nfor beads (else Chemyx)"() -> (w2601:bool)
        n1699 = disable-structure shown="Disabled" {
          disable-tunnel: w2601 -> [w2603 _]
          disable-tunnel: w2600 -> [w2602 _]
          frame Disabled {
            n1700 = case shown="True" w2603 {
              tunnel: "Inject Pump 3" -> [w2607 w2648]
              tunnel: w2602 -> [_ w2649]
              frame False {
                n1701 = local read "Pump write delay (ms)"() -> (w2606:dbl)
                n1702 = case shown="True" w2607 {
                  tunnel: w2606 -> [w2613 w2627]
                  tunnel: "Chemyx Syringe Pump Serial Port" -> [w2610 w2626]
                  frame False {
                    n1703 = flat-sequence {
                      tunnel: w2610 -> [w2614]
                      tunnel: [w2614] -> w2611
                      tunnel: w2613 -> [_]
                      tunnel: [w2617] -> w2612
                      tunnel: w2611 -> [w2617]
                      tunnel: w2612 -> [w2618]
                      tunnel: [w2618] -> w2608
                      tunnel: [w2620] -> w2609
                      tunnel: w2608 -> [w2620]
                      tunnel: w2609 -> [w2622]
                      frame #0 {
                        n1704 = call "Write to pump.vi"("string"="enter pump3", "VISA resource name"=w2614) -> ()  [unwired: 1 out]
                      }
                      frame #1 {
                        n1705 = local read "Pump pause delay (ms)"() -> (w2616:u32)
                        n1706 = Wait (ms)(milliseconds to wait=w2616) -> ()  [unwired: 1 out]
                      }
                      frame #2 {
                        n1707 = call "Write to pump.vi"("string"="stop", "VISA resource name"=w2618) -> ()  [unwired: 1 out]
                      }
                      frame #3 {
                        n1708 = Wait (ms)(milliseconds to wait=u32 0) -> ()  [unwired: 1 out]
                      }
                      frame #4 {
                        n1709 = call "Write to pump.vi"("string"="stop", "VISA resource name"=w2622) -> ()  [unwired: 1 out]
                      }
                    }
                  }
                  frame True {
                    n1710 = flat-sequence {
                      tunnel: w2626 -> [w2636]
                      tunnel: w2627 -> [w2631]
                      tunnel: w2627 -> [w2638]
                      tunnel: w2626 -> [w2639]
                      tunnel: [w2639] -> w2625
                      tunnel: [w2642] -> w2624
                      tunnel: w2625 -> [w2642]
                      tunnel: w2624 -> [w2643]
                      frame #0 {
                        n1711 = local read "All Pump Parameters"() -> (w2630:T10)
                        n1712 = Unbundle By Name(w2630) -> ("Pump 3"=w2637:T49)
                        n1713 = call "Set pump parameters.vi"("Pump write delay (ms)"=w2631, "Volume (uL)"="Ch 3 Inject Volume (uL)", "Rate (uL/h)"="Ch 3 Inject Rate (ul/h)", "Units"=4.0, "Pump #"=3.0, "Pump Parameters In"=w2637, "VISA resource name"=w2636) -> ("Pump Parameters Out"=w2629:T49)  [unwired: 3 in]
                        n1714 = Bundle By Name(cluster=w2630, "Pump 3"=w2629) -> (w2628:T10)
                        n1715 = local write "All Pump Parameters"(w2628) -> ()
                      }
                      frame #1 {
                        n1716 = Wait (ms)(milliseconds to wait=w2638) -> ()  [unwired: 1 out]
                      }
                      frame #2 {
                        n1717 = call "Write to pump.vi"("string"="start", "VISA resource name"=w2639) -> ()  [unwired: 1 out]
                      }
                      frame #3 {
                        n1718 = Wait (ms)(milliseconds to wait=u32 500) -> ()  [unwired: 1 out]
                      }
                      frame #4 {
                        n1719 = call "Write to pump.vi"("string"="start", "VISA resource name"=w2643) -> ()  [unwired: 1 out]
                      }
                    }
                  }
                }
              }
              frame True {
                n1720 = case shown="False" w2648 {
                  tunnel: w2649 -> [w2661 w2668]
                  frame False {
                    n1721 = flat-sequence {
                      tunnel: w2661 -> [w2663]
                      frame #0 {
                        n1722 = local write "Flushing P3"(FALSE ("Flushing P3")) -> ()
                        n1723 = Concatenate Strings("stop" ("string"), "\r") -> (w2665:string)
                        n1724 = VISA Write(VISA resource name=w2663, write buffer=w2665) -> ()  [unwired: 1 in, 3 out]
                      }
                      frame #1 {
                        n1725 = property on="Clear Volume P3" class="Bool (strict)"("Val(Sgnl)"=TRUE ("Value (Signaling)")) -> ()  [unwired: 2 in, 2 out]
                      }
                    }
                  }
                  frame True {
                    n1726 = local read "Normal Flow Rate (ul/h) P3"() -> (w2669:dbl)
                    n1727 = Number To Decimal String(number=w2669) -> (decimal integer string=w2675:string)  [unwired: 1 in]
                    n1728 = Concatenate Strings("irate  " ("string"), w2675, " u/h" ("string"), "\r") -> (w2673:string)
                    n1729 = VISA Write(VISA resource name=w2668, write buffer=w2673) -> (VISA resource name out=w2671:refnum<visa-resource-name>)  [unwired: 1 in, 2 out]
                    n1730 = Concatenate Strings("irun" ("string"), "\r") -> (w2677:string)
                    n1731 = VISA Write(VISA resource name=w2671, write buffer=w2677) -> ()  [unwired: 1 in, 3 out]
                  }
                }
                n1732 = local read "Save Event Log?"() -> (w2646:bool)
                n1733 = local read "Saving..."() -> (w2647:bool)
                n1734 = And(x=w2647, y=w2646) -> (x .and. y?=w2645:bool)
                n1735 = case shown="True" w2645 {
                  tunnel: w2648 -> [_ w2656]
                  frame False {
                  }
                  frame True {
                    n1736 = local read "Normal Flow Rate (ul/h) P3"() -> (w2650:dbl)
                    n1737 = Number To Decimal String(number=w2650) -> (decimal integer string=w2652:string)  [unwired: 1 in]
                    n1738 = Concatenate Strings("on, flow rate", w2652) -> (w2651:string)
                    n1739 = local read "log file ref"() -> (w2655:refnum<file>)
                    n1740 = Select(t=w2651, s=w2656, f="off") -> (s? t:f=w2657:string)
                    n1741 = local read "Time (s)"() -> (w2654:dbl)
                    n1742 = Concatenate Strings("pump 3 ", w2657) -> (w2659:string)
                    n1743 = call "write to event log.vi"("log file ref"=w2655, "time"=w2654, "input string"=w2659) -> ()  [unwired: 8 in]
                  }
                }
              }
            }
          }
          frame Enabled {
          }
        }
      }
      event "Inject Pump 2": Value Change {
        n1744 = event-data() -> ()  [unwired: 7 out]
        n1745 = local read "Pump write delay (ms)"() -> (w2684:dbl)
        n1746 = local read "Chemyx Syringe Pump Serial Port"() -> (w2683:refnum<visa-resource-name>)
        n1747 = flat-sequence {
          tunnel: w2683 -> [w2708]
          tunnel: w2684 -> [w2704]
          tunnel: "Inject Pump 2" -> [_]
          tunnel: w2684 -> [w2710]
          tunnel: w2683 -> [w2711]
          frame #0 {
            n1748 = local read "All Pump Parameters"() -> (w2703:T10)
            n1749 = Multiply(x=60.0, y="Flush Center Ch Rate (ul/m)") -> (x*y=w2700:dbl)
            n1750 = Unbundle By Name(w2703) -> ("Pump 2"=w2709:T49)
            n1751 = call "Set pump parameters.vi"("Pump write delay (ms)"=w2704, "Volume (uL)"="Flush Center Ch Volume (uL)", "Rate (uL/h)"=w2700, "Units"=3.0, "Pump #"=2.0, "Pump Parameters In"=w2709, "VISA resource name"=w2708) -> ("Pump Parameters Out"=w2702:T49)  [unwired: 3 in]
            n1752 = Bundle By Name(cluster=w2703, "Pump 2"=w2702) -> (w2701:T10)
            n1753 = local write "All Pump Parameters"(w2701) -> ()
            n1754 = Add(x="Flush Center Ch Volume (uL)", y="Total Volume\nFlushed (uL)") -> (x+y=w2697:dbl)
            n1755 = local write "Total Volume\nFlushed (uL)"(w2697) -> ()
          }
          frame #1 {
            n1756 = Wait (ms)(milliseconds to wait=w2710) -> ()  [unwired: 1 out]
          }
          frame #2 {
            n1757 = call "Write to pump.vi"("string"="start", "VISA resource name"=w2711) -> ()  [unwired: 1 out]
          }
        }
        n1758 = local read "Save Event Log?"() -> (w2682:bool)
        n1759 = local read "Saving..."() -> (w2681:bool)
        n1760 = And(x=w2682, y=w2681) -> (x .and. y?=w2680:bool)
        n1761 = case shown="True" w2680 {
          tunnel: "Inject Pump 2" -> [_ w2691]
          frame False {
          }
          frame True {
            n1762 = local read "Flow rate (uL/h)"() -> (w2685:dbl)
            n1763 = Number To Decimal String(number=w2685) -> (decimal integer string=w2687:string)  [unwired: 1 in]
            n1764 = Concatenate Strings("on, flow rate", w2687) -> (w2686:string)
            n1765 = Select(t=w2686, s=w2691, f="off") -> (s? t:f=w2695:string)
            n1766 = local read "Time (s)"() -> (w2689:dbl)
            n1767 = local read "log file ref"() -> (w2690:refnum<file>)
            n1768 = Concatenate Strings("pump 2 ", w2695) -> (w2693:string)
            n1769 = call "write to event log.vi"("log file ref"=w2690, "time"=w2689, "input string"=w2693) -> ()  [unwired: 8 in]
          }
        }
      }
      event "Sample Channel\nFlow": Value Change {
        n1770 = event-data() -> ()  [unwired: 7 out]
        n1771 = disable-structure shown="Disabled" {
          disable-tunnel: w2713 -> [w2720 _]
          frame Disabled {
            n1772 = Select(t="irun" ("string"), s="Sample Channel\nFlow", f="stop" ("string")) -> (s? t:f=w2715:string)
            n1773 = Concatenate Strings(w2715, "\r") -> (w2718:string)
            n1774 = VISA Write(VISA resource name=w2720, write buffer=w2718) -> ()  [unwired: 1 in, 3 out]
          }
          frame Enabled {
          }
        }
      }
      event "Start Flow": Value Change {
        n1775 = event-data() -> ()  [unwired: 7 out]
        n1776 = disable-structure shown="Disabled" {
          disable-tunnel: w2721 -> [w2722 _]
          frame Disabled {
            n1777 = local write "Sample Channel\nFlow"(TRUE ("Sample Channel\nFlow")) -> ()
            n1778 = local write "Start Flow"(FALSE ("Start Flow")) -> ()
            n1779 = Concatenate Strings("irun" ("string"), "\r") -> (w2726:string)
            n1780 = VISA Write(VISA resource name=w2722, write buffer=w2726) -> ()  [unwired: 1 in, 3 out]
          }
          frame Enabled {
          }
        }
      }
      event "Stop Flow": Value Change {
        n1781 = event-data() -> ()  [unwired: 7 out]